vi "IR Opo Main.vi"() -> ()   [LabVIEW 2016] (continued)
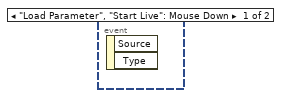
[diagram p2: hidden frame]
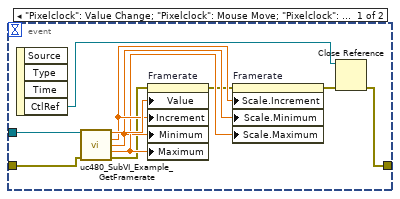
[diagram p3: hidden frame]
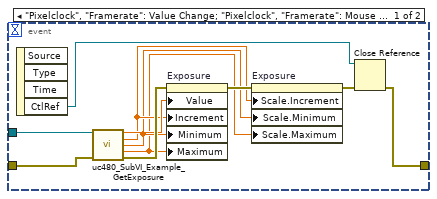
[diagram p4: hidden frame]
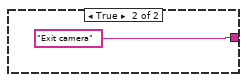
[diagram p5: hidden frame]
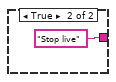
[diagram p6: hidden frame]
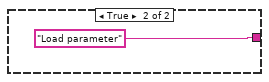
[diagram p7: hidden frame]
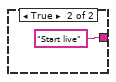
[diagram p8: hidden frame]
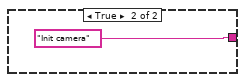
[diagram p9: hidden frame]
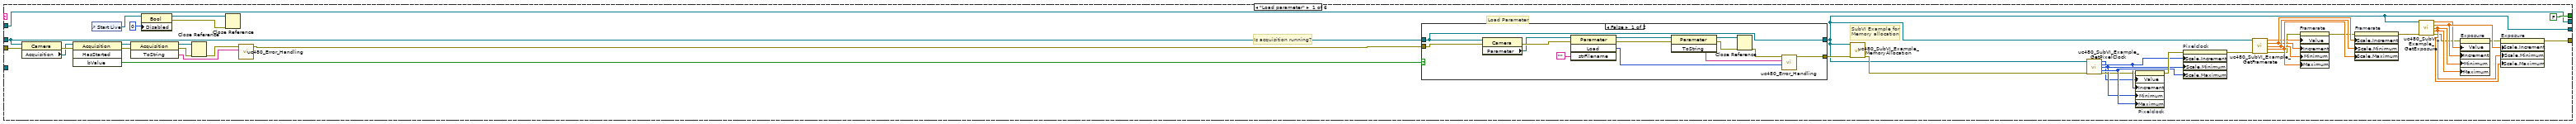
[diagram p10: hidden frame]
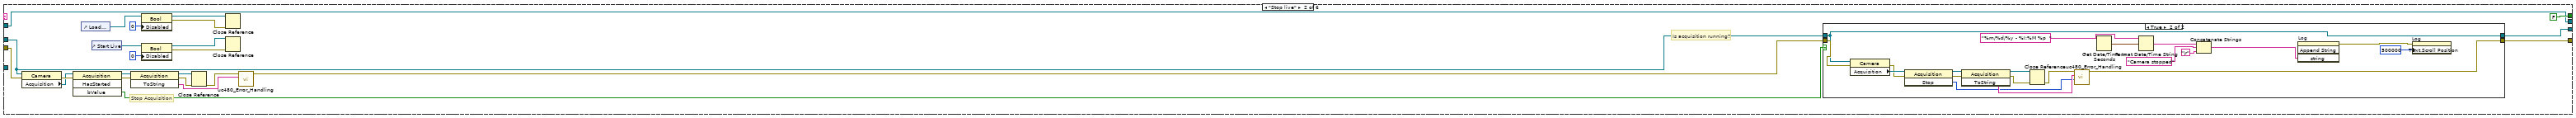
[diagram p12: hidden frame]
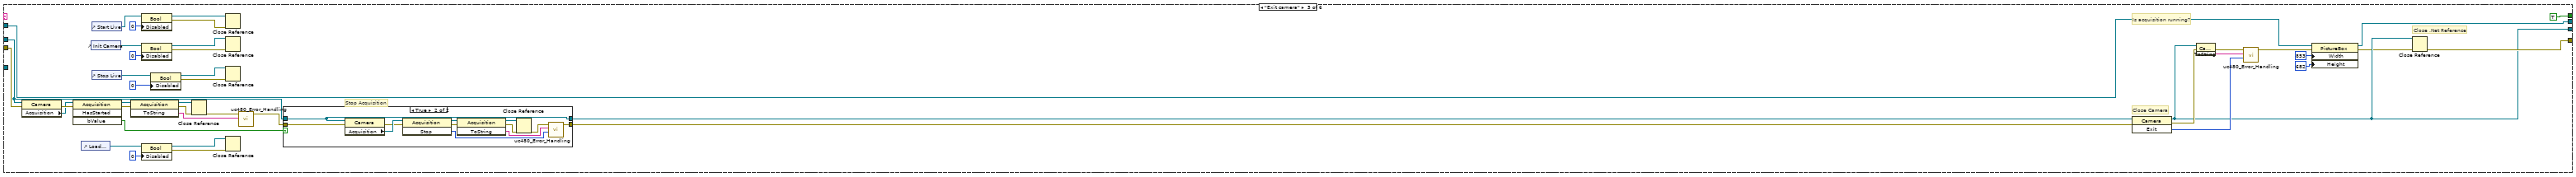
[diagram p14: hidden frame]
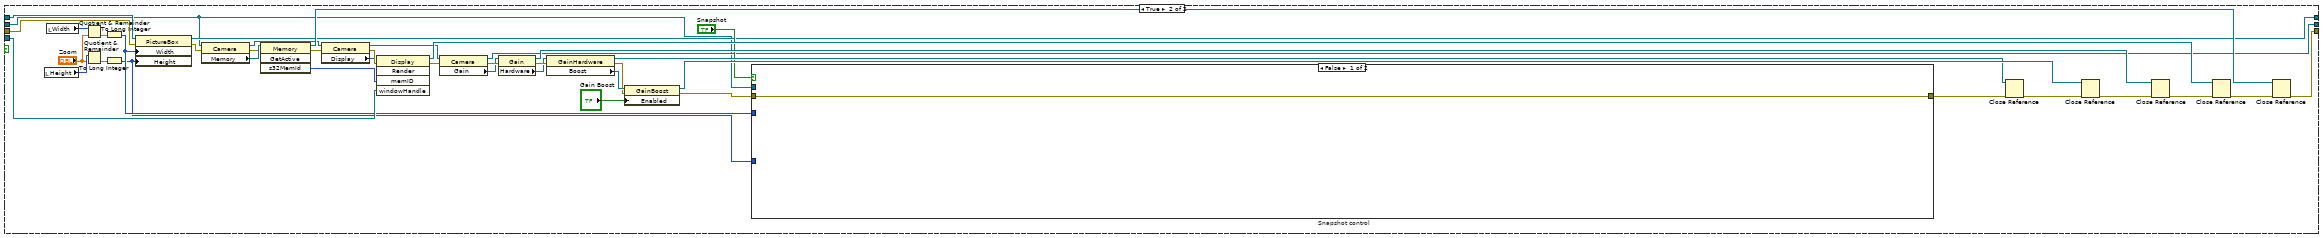
[diagram p16: hidden frame]
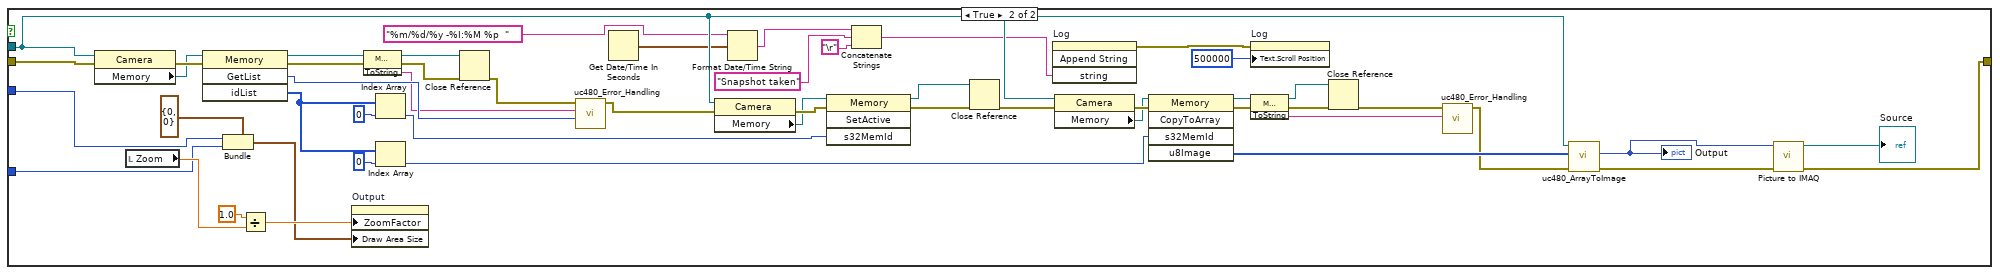
[diagram p17: hidden frame]
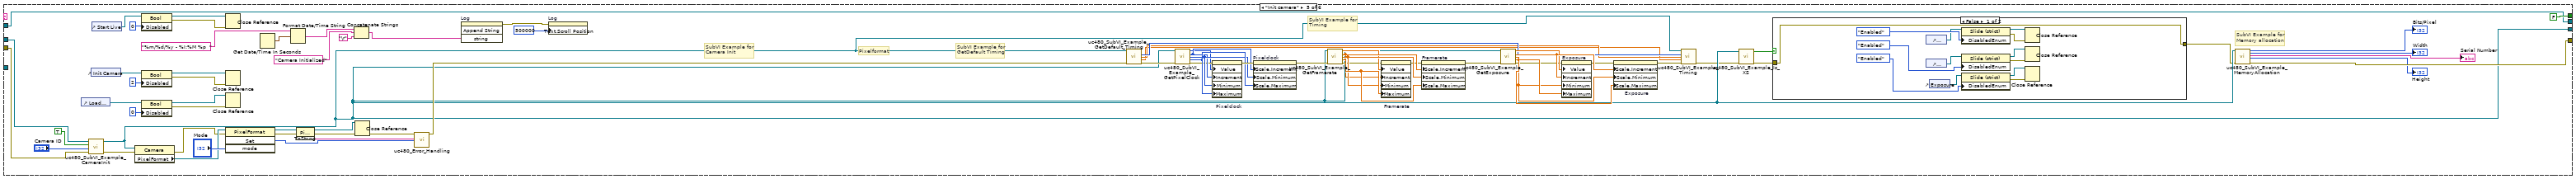
[diagram p18: hidden frame]
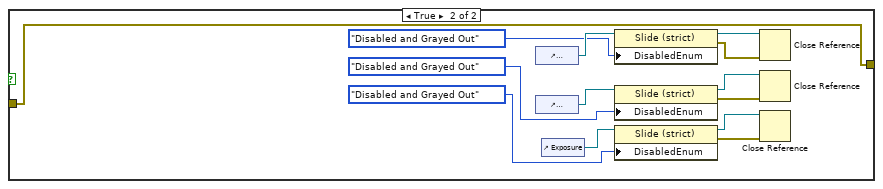
[diagram p19: hidden frame]
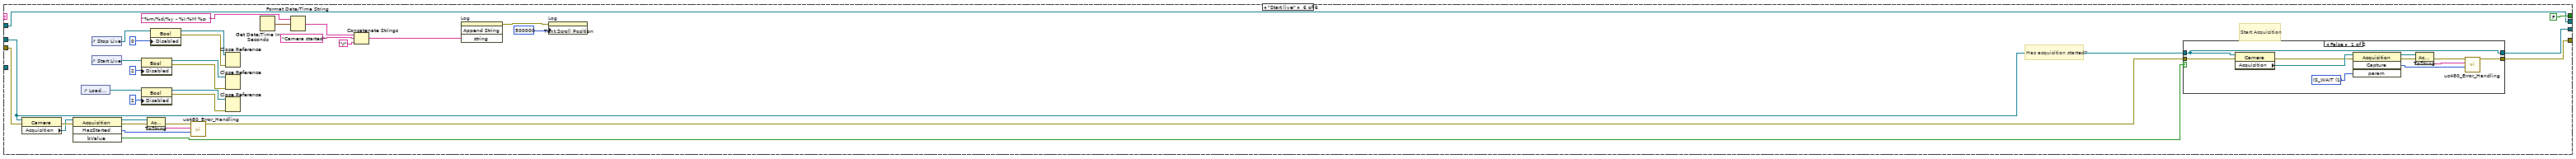
[diagram p20: hidden frame]
            n536 = local read "Y offset"() -> (w1451:i32)
            n537 = call <vilib>:"Simple Error Handler.vi"("error in (no error)"=w1382) -> ()  [unwired: 4 in, 5 out]
            n538 = Unbundle(w1387) -> ("Global Rectangle[0]"=w1386:i32, "Global Rectangle[1]"=w1385:i32)
            n539 = Empty Array?(array=w1437) -> (empty?=w1438:bool)
            n540 = Subtract(x=w1386, y=w1450) -> (x-y=w1457:i32)
            n541 = Subtract(x=w1385, y=w1451) -> (x-y=w1456:i32)
            n542 = case shown="False" w1438 {
              tunnel: [w1478 u8[][] [[1]] ("Image Pixels (U8)")] -> w1436
              tunnel: w1437 -> [w1478 _]
              frame False {
              }
              frame True {
                n543 = One Button Dialog(message="ATTENTION: you did not select\nany region of interest") -> ()  [unwired: 1 in, 1 out]
              }
            }
            n544 = local read "Heigth (µm)"() -> (w1421:i32)
            n545 = local read "Width (µm)"() -> (w1420:i32)
            n546 = Divide "X spot radius in micron"(x=w1420, y=w1415) -> (x/y=w1424:dbl)
            n547 = Divide "Y spot radius in micron"(x=w1421, y=w1415) -> (x/y=w1423:dbl)
            n548 = local read "Pixel size"() -> (w1389:dbl)
            n549 = Divide "X spot diameter in pixel"(x=w1420, y=w1389) -> (x/y=w1393:dbl)
            n550 = Divide "Y spot diameter in pixel"(x=w1421, y=w1389) -> (x/y=w1394:dbl)
            n551 = Multiply(x=w1389, y=w1389) -> (x*y=w1441:dbl)
            n552 = Multiply(x=w1457, y=w1389) -> (x*y=w1417:dbl)
            n553 = Multiply(x=w1456, y=w1389) -> (x*y=w1425:dbl)
            n554 = Round To Nearest(number=w1424) -> (nearest integer value=w1418:dbl)
            n555 = Round To Nearest(number=w1423) -> (nearest integer value=w1419:dbl)
            n556 = Add(x=w1417, y=w1418) -> (x+y=w1416:dbl)
            n557 = Add(x=w1425, y=w1419) -> (x+y=w1422:dbl)
            n558 = To Double Precision Float(number=w1436) -> (double precision float=w1439:dbl[][])
            n559 = Array Size(array=w1436) -> (size(s)=w1461:i32[])
            n560 = local read "Height  step \ndivider"() -> (w1463:i32)
            n561 = Divide(x=w1416, y=w1447) -> (x/y=w1449:dbl)
            n562 = Divide(x=w1422, y=w1447) -> (x/y=w1448:dbl)
            n563 = Add Array Elements(numeric array=w1439) -> (sum=w1443:dbl)
            n564 = Array To Cluster(array=w1461) -> (cluster=w1462:cluster{"[0]":i32, "[1]":i32})
            n565 = Number To Fractional String(number=w1449, precision (6)=w1455) -> (F-format string=w1434:string)  [unwired: 2 in]
            n566 = Number To Fractional String(number=w1448, precision (6)=w1455) -> (F-format string=w1435:string)  [unwired: 2 in]
            n567 = Unbundle(w1462) -> ("[0]"=w1381:i32, "[1]"=w1397:i32)
            n568 = Divide(x=w1443, y=u8 255) -> (x/y=w1440:dbl)
            n569 = Multiply "# pixels in an ablation spot"(x=w1394, y=w1393) -> (x*y=w1396:dbl)
            n570 = Multiply(x=w1440, y=w1441) -> (x*y=w1431:dbl)
            n571 = Multiply(x=w1381, y=w1389) -> (x*y=w1427:dbl)
            n572 = Multiply(x=w1397, y=w1389) -> (x*y=w1428:dbl)
            n573 = Subtract(x=w1397, y=w1393) -> (x-y=w1414:dbl)
            n574 = Fract/Exp String To Number(string=w1434) -> (number=→"Axis 1 Offset":dbl)  [unwired: 3 in, 1 out]
            n575 = Fract/Exp String To Number(string=w1435) -> (number=→"Axis 2 Offset":dbl)  [unwired: 3 in, 1 out]
            n576 = Divide "Height of a line"(x=w1394, y=w1463) -> (x/y=w1391:dbl)
            n577 = Divide "Total heigth lines"(x=w1381, y=w1391) -> (x/y=w1395:dbl)
            n578 = Multiply(x=w1389, y=w1391) -> (x*y=w1392:dbl)
            n579 = Round To Nearest(number=w1427) -> (nearest integer value=→"ROI container\nheigth (µm)":dbl)
            n580 = Round To Nearest(number=w1428) -> (nearest integer value=→"ROI container\nwidth (µm)":dbl)
            n581 = Divide(x=w1431, y=1000000.0) -> (x/y=→"ROI Area \n(mm2)":dbl)
            n582 = Divide(x="Precision (%)", y=100.0) -> (x/y=w1380:dbl)
            n583 = call "ROI parser.vi"("# pixels in an ablation spot"=w1396, "ROI Height in pixel"=w1395, "Heigth step size in pixel"=w1391, "ROI (8 bit image)"=w1436, "Ablation spot width"=w1393, "ROI Width in pixel"=w1414, "Sampling\nPrecision"=w1380, "Ablation spot heigth"=w1394) -> ("Parsed array"=w1476:bool[][])  [unwired: 3 in]
            n584 = Index Array(array=w1476, index (col)=0 ("disabled index (col)")) -> (element=w1474:bool[])  [unwired: 1 in]
            n585 = Array Size(array=w1474) -> (size(s)=w1475:i32)
            n586 = call "Array processor.vi"("Source array"=w1476, "Iterations"=w1475) -> ("Lenght product array"=w1473:i32[][], "T/F product array"=w1410:bool[][])  [unwired: 8 in]
            n587 = for {
              tunnel: w1473 -> [w1486] mode=indexing
              tunnel: [w1485] -> w1459 mode=indexing
              tunnel: w1389 -> [w1484]
              # "This loop transform each lenght fragment into a µm size value"
              n588 = Multiply(x=w1484, y=w1486) -> (x*y=w1485:dbl[])
            }
            n589 = Array Size(array=w1410) -> (size(s)=w1409:i32[])
            n590 = Index Array(array=w1410, index (col)=0 ("disabled index (col)")) -> (element=w1465:bool[])  [unwired: 1 in]
            n591 = Array Size(array=w1465) -> (size(s)=w1464:i32)
            n592 = Index Array(array=w1409, index=0) -> (element=w1406:i32)
            n593 = Index Array(array=w1409, index=1) -> (element=w1405:i32)
            n594 = for {
              N: w1464 -> [_]
              tunnel: w1410 -> [w1483] mode=indexing
              tunnel: [w1481] -> w1446 mode=indexing
              # "This loop add a F for each Y moviment"
              n595 = Build Array (concatenate)(w1483, FALSE) -> (w1481:bool[])
            }
            "Laser on/off array" <- w1446
            n596 = Multiply(x=w1406, y=w1405) -> (x*y=w1404:i32)
            n597 = Multiply(x=w1404, y=w1403) -> (x*y=w1402:dbl)
            n598 = Round To Nearest(number=w1392) -> (nearest integer value=w1390:dbl)
            n599 = local read "Speed (µm/s)"() -> (w1411:i32)
            n600 = Index Array(array=w1459, index (col)=0 ("disabled index (col)")) -> (element=w1469:dbl[])  [unwired: 1 in]
            n601 = Index Array(array=w1459, index (row)=0) -> (element=w1471:dbl[])  [unwired: 1 in]
            n602 = Array Size(array=w1469) -> (size(s)=w1467:i32)
            n603 = Array Size(array=w1471) -> (size(s)=w1470:i32)
            n604 = local read "Axis 1"() -> (w1413:string)
            n605 = local read "Axis 2"() -> (w1412:string)
            n606 = call "Commands array generator.vi"("Axis 1"=w1413, "Heigth"=w1467, "Axis in"=w1412, "Width"=w1470, "Axes speed \n(µm/s)"=w1411, "Y Step size in µm"=w1390, "T/F product array"=w1410, "Space defined array"=w1459) -> ("Command Array"=→"Commands array":string[][], "Time Array"=w1426:dbl[][])  [unwired: 2 in]
            "Time array" <- w1426
            n607 = Add Array Elements(numeric array=w1426) -> (sum=w1401:dbl)
            n608 = Add(x=w1402, y=w1401) -> (x+y=w1400:dbl)
            "Processi time (sec)" <- w1400
            n609 = local write "Process time"(w1400) -> ()
          }
        }
      }
      event "Axes Manual Control": Value Change {
        n610 = event-data() -> ()  [unwired: 1 in, 6 out]
        n611 = case shown="True" "Axes Manual Control" {
          tunnel: w1489 -> [_ w1501]
          tunnel: w1488 -> [_ w1500]
          tunnel: w1487 -> [_ w1499]
          frame False {
          }
          frame True {
            n612 = flat-sequence {
              tunnel: w1501 -> [w1511]
              tunnel: w1500 -> [w1510]
              tunnel: w1499 -> [w1509]
              tunnel: [w1511] -> w1498
              tunnel: [w1510] -> w1497
              tunnel: [w1509] -> w1496
              tunnel: [w1508] -> w1495
              tunnel: [w1507] -> w1494
              tunnel: [w1506] -> w1493
              tunnel: [w1505] -> w1492
              tunnel: w1498 -> [w1554]
              tunnel: w1497 -> [w1553]
              tunnel: w1496 -> [w1552]
              tunnel: w1495 -> [w1547]
              tunnel: w1494 -> [w1546]
              tunnel: w1493 -> [w1537]
              tunnel: w1492 -> [w1536]
              frame #0 {
                n613 = call <userlib>:"Open TCP-IP.vi"("IP address"=w1511) -> ("error out"=w1503:errorcluster, "Connection ID"=w1512:T6)  [unwired: 8 in, 1 out]
                n614 = call <vilib>:"Simple Error Handler.vi"("error in (no error)"=w1503) -> ("error?"=w1502:bool, "error out"=w1504:errorcluster)  [unwired: 4 in, 3 out]
                n615 = case shown="True" w1502 {
                  tunnel: w1512 -> [w1527 _]
                  tunnel: w1504 -> [w1526 _]
                  tunnel: w1510 -> [w1523 _]
                  tunnel: w1509 -> [w1522 _]
                  tunnel: [w1521 w1531] -> w1508
                  tunnel: [w1520 w1531] -> w1507
                  tunnel: [w1516 w1530] -> w1506
                  tunnel: [w1515 w1530] -> w1505
                  frame False {
                    n616 = call "Get Stages Status.vi"("error in (no error)"=w1526, "Group Name (250 c max)"=w1523, "connection ID in"=w1527) -> ("error out"=w1525:errorcluster, "XPS error out"=w1524:errorcluster, "Group Status String"=w1520:string, "connection ID out"=w1519:T6, "Status"=w1515:i32)  [unwired: 4 in]
                    n617 = call "Get Stages Status.vi"("error in (no error)"=w1525, "XPS error in (no error)"=w1524, "Group Name (250 c max)"=w1522, "connection ID in"=w1519) -> ("error out"=w1529:errorcluster, "XPS error out"=w1518:errorcluster, "Group Status String"=w1521:string, "connection ID out"=w1528:T6, "Status"=w1516:i32)  [unwired: 3 in]
                    n618 = call <vilib>:"Simple Error Handler.vi"("error source (\" \")"="Axis manual control check" ("error source (\" \")"), "error in (no error)"=w1518) -> ()  [unwired: 3 in, 5 out]
                    n619 = call <userlib>:"Close TCP-IP.vi"("error in (no error)"=w1529, "connection ID in"=w1528) -> ("Error out"=w1517:errorcluster)  [unwired: 9 in]
                    n620 = call <vilib>:"Simple Error Handler.vi"("error source (\" \")"="TCP close Axis manual control check" ("error source (\" \")"), "error in (no error)"=w1517) -> ()  [unwired: 3 in, 5 out]
                  }
                  frame True {
                    w1530 = 0
                    w1531 = ""
                  }
                }
              }
              frame #1 {
                w1540 = 47 ("y")
                w1541 = "Ready"
                n621 = String Subset(string=w1546, offset (0)=0, length (rest)=5 ("length (rest)")) -> (substring=w1543:string)
                n622 = String Subset(string=w1547, offset (0)=0, length (rest)=5 ("length (rest)")) -> (substring=w1542:string)
                n623 = Equal?(x=w1543, y=w1541) -> (x = y?=w1544:bool)
                n624 = Equal?(x=w1541, y=w1542) -> (x = y?=w1545:bool)
                n625 = Equal?(x=w1540, y=w1536) -> (x = y?=w1538:bool)
                n626 = Equal?(x=w1537, y=w1540) -> (x = y?=w1539:bool)
                n627 = And(x=w1539, y=w1538) -> (x .and. y?=w1533:bool)
                n628 = And(x=w1544, y=w1545) -> (x .and. y?=w1534:bool)
                n629 = Not(x=w1533) -> (.not. x?=w1532:bool)
                n630 = And(x=w1534, y=w1532) -> (x .and. y?=w1535:bool)
                n631 = case shown="True" w1535 {
                  tunnel: w1554 -> [_ w1560]
                  tunnel: w1553 -> [_ w1559]
                  tunnel: w1552 -> [_ w1558]
                  tunnel: w1532 -> [w1555 _]
                  frame False {
                    n632 = case shown="False" w1555 {
                      frame False {
                        n633 = One Button Dialog(message="One or more axis already in jogging position") -> ()  [unwired: 1 in, 1 out]
                      }
                      frame True {
                        n634 = One Button Dialog(message="Axes are not ready") -> ()  [unwired: 1 in, 1 out]
                      }
                    }
                  }
                  frame True {
                    n635 = call "XPS_LTA_HS_Jogger.vi"("Axis 2"=w1558, "Axis 1"=w1559, "Controller Address"=w1560) -> ()  [unwired: 8 in]
                  }
                }
              }
            }
          }
        }
      }
      event "Home Axes": Value Change {
        n636 = event-data() -> ()  [unwired: 1 in, 6 out]
        n637 = flat-sequence {
          tunnel: w1567 -> [w1573]
          tunnel: w1568 -> [w1574]
          tunnel: w1569 -> [w1575]
          tunnel: "Home Axes" -> [w1576]
          tunnel: [w1576] -> w1565
          tunnel: [w1575] -> w1564
          tunnel: [w1574] -> w1563
          tunnel: [w1573] -> w1562
          tunnel: [w1572] -> w1561
          tunnel: [w1580] -> w1566
          tunnel: w1565 -> [w1578]
          tunnel: w1564 -> [w1583]
          tunnel: w1563 -> [w1581]
          tunnel: w1562 -> [w1582]
          tunnel: w1561 -> [w1579]
          tunnel: [w1662] -> w1570
          tunnel: w1566 -> [w1661]
          frame #0 {
            n638 = call "Display Message to User"() -> ("OK"=w1572:bool)  [unwired: 10 in, 1 out]
          }
          frame #1 {
            n639 = And(x=w1578, y=w1579) -> (x .and. y?=w1577:bool)
            n640 = case shown="True" w1577 {
              tunnel: w1583 -> [_ w1599]
              tunnel: w1581 -> [_ w1600]
              tunnel: w1582 -> [_ w1597]
              tunnel: w1581 -> [_ w1598]
              tunnel: [FALSE w1590] -> w1580
              frame False {
              }
              frame True {
                w1596 = 47 ("y")
                w1612 = "Ready"
                n641 = call <userlib>:"Open TCP-IP.vi"("IP address"=w1599) -> ("error out"=w1585:errorcluster, "Connection ID"=w1603:T6)  [unwired: 8 in, 1 out]
                n642 = call <vilib>:"Simple Error Handler.vi"("error in (no error)"=w1585) -> ("error?"=w1587:bool, "error out"=w1586:errorcluster)  [unwired: 4 in, 3 out]
                n643 = case shown="True" w1587 {
                  tunnel: w1586 -> [w1626 _]
                  tunnel: w1603 -> [w1625 _]
                  tunnel: [w1622 w1631] -> w1602
                  tunnel: [w1621 w1631] -> w1601
                  tunnel: w1600 -> [w1620 _]
                  tunnel: w1597 -> [w1619 _]
                  tunnel: [w1616 w1630] -> w1595
                  tunnel: [w1615 w1630] -> w1594
                  frame False {
                    n644 = call "Get Stages Status.vi"("error in (no error)"=w1626, "Group Name (250 c max)"=w1620, "connection ID in"=w1625) -> ("error out"=w1627:errorcluster, "XPS error out"=w1628:errorcluster, "Group Status String"=w1622:string, "connection ID out"=w1629:T6, "Status"=w1615:i32)  [unwired: 4 in]
                    n645 = call "Get Stages Status.vi"("error in (no error)"=w1627, "XPS error in (no error)"=w1628, "Group Name (250 c max)"=w1619, "connection ID in"=w1629) -> ("error out"=w1623:errorcluster, "XPS error out"=w1618:errorcluster, "Group Status String"=w1621:string, "connection ID out"=w1624:T6, "Status"=w1616:i32)  [unwired: 3 in]
                    n646 = call <vilib>:"Simple Error Handler.vi"("error source (\" \")"="home axis check" ("error source (\" \")"), "error in (no error)"=w1618) -> ()  [unwired: 3 in, 5 out]
                    n647 = call <userlib>:"Close TCP-IP.vi"("error in (no error)"=w1623, "connection ID in"=w1624) -> ("Error out"=w1617:errorcluster)  [unwired: 9 in]
                    n648 = call <vilib>:"Simple Error Handler.vi"("error source (\" \")"="TCP close home axis check" ("error source (\" \")"), "error in (no error)"=w1617) -> ()  [unwired: 3 in, 5 out]
                  }
                  frame True {
                    w1630 = 0
                    w1631 = ""
                  }
                }
                n649 = Equal?(x=w1596, y=w1594) -> (x = y?=w1593:bool)
                n650 = Equal?(x=w1595, y=w1596) -> (x = y?=w1592:bool)
                n651 = String Subset(string=w1602, offset (0)=0, length (rest)=5 ("length (rest)")) -> (substring=w1610:string)
                n652 = String Subset(string=w1601, offset (0)=0, length (rest)=5 ("length (rest)")) -> (substring=w1611:string)
                n653 = Equal?(x=w1610, y=w1612) -> (x = y?=w1609:bool)
                n654 = Equal?(x=w1612, y=w1611) -> (x = y?=w1608:bool)
                n655 = And(x=w1592, y=w1593) -> (x .and. y?=w1588:bool)
                n656 = Not(x=w1588) -> (.not. x?=w1589:bool)
                n657 = And(x=w1609, y=w1608) -> (x .and. y?=w1591:bool)
                n658 = And(x=w1591, y=w1589) -> (x .and. y?=w1590:bool)
                n659 = case shown="True" w1590 {
                  tunnel: w1599 -> [_ w1641]
                  tunnel: w1598 -> [_ w1640]
                  tunnel: w1597 -> [_ w1639]
                  tunnel: w1588 -> [w1632 _]
                  frame False {
                    n660 = case shown="True" w1632 {
                      frame False {
                        n661 = One Button Dialog(message="Axes are not ready") -> ()  [unwired: 1 in, 1 out]
                      }
                      frame True {
                        n662 = One Button Dialog(message="One or more axis are in jogging mode") -> ()  [unwired: 1 in, 1 out]
                      }
                    }
                  }
                  frame True {
                    n663 = call <userlib>:"Open TCP-IP.vi"("IP address"=w1641) -> ("error out"=w1657:errorcluster, "Connection ID"=w1658:T6)  [unwired: 8 in, 1 out]
                    n664 = call <userlib>:"Group Kill.vi"("error in (no error)"=w1657, "Group Name (250 c max)"=w1640, "connection ID in"=w1658) -> ("error out"=w1655:errorcluster, "XPS error out"=w1656:errorcluster, "connection ID out"=w1652:T6)  [unwired: 6 in]
                    n665 = call <userlib>:"Group Initialize.vi"("error in (no error)"=w1655, "XPS error in (no error)"=w1656, "Group Name (250 c max)"=w1640, "connection ID in"=w1652) -> ("error out"=w1653:errorcluster, "XPS error out"=w1654:errorcluster, "connection ID out"=w1651:T6)  [unwired: 5 in]
                    n666 = call <userlib>:"Group Home Search.vi"("error in (no error)"=w1653, "XPS error in (no error)"=w1654, "Group Name (250 c max)"=w1640, "connection ID in"=w1651) -> ("error out"=w1642:errorcluster, "XPS error out"=w1643:errorcluster, "connection ID out"=w1650:T6)  [unwired: 5 in]
                    n667 = call <userlib>:"Group Kill.vi"("error in (no error)"=w1642, "XPS error in (no error)"=w1643, "Group Name (250 c max)"=w1639, "connection ID in"=w1650) -> ("error out"=w1644:errorcluster, "XPS error out"=w1645:errorcluster, "connection ID out"=w1649:T6)  [unwired: 5 in]
                    n668 = call <userlib>:"Group Initialize.vi"("error in (no error)"=w1644, "XPS error in (no error)"=w1645, "Group Name (250 c max)"=w1639, "connection ID in"=w1649) -> ("error out"=w1646:errorcluster, "XPS error out"=w1647:errorcluster, "connection ID out"=w1648:T6)  [unwired: 5 in]
                    n669 = call <userlib>:"Group Home Search.vi"("error in (no error)"=w1646, "XPS error in (no error)"=w1647, "Group Name (250 c max)"=w1639, "connection ID in"=w1648) -> ("error out"=w1659:errorcluster, "XPS error out"=w1638:errorcluster, "connection ID out"=w1660:T6)  [unwired: 5 in]
                    n670 = call <vilib>:"Simple Error Handler.vi"("error source (\" \")"="home axis " ("error source (\" \")"), "error in (no error)"=w1638) -> ()  [unwired: 3 in, 5 out]
                    n671 = call <userlib>:"Close TCP-IP.vi"("error in (no error)"=w1659, "connection ID in"=w1660) -> ("Error out"=w1637:errorcluster)  [unwired: 9 in]
                    n672 = call <vilib>:"Simple Error Handler.vi"("error source (\" \")"="TCP close home axis " ("error source (\" \")"), "error in (no error)"=w1637) -> ()  [unwired: 3 in, 5 out]
                  }
                }
              }
            }
          }
          frame #2 {
            n673 = case shown="True" w1661 {
              tunnel: ["" ("StringOut") "Axes have been moved to home position" ("StringOut")] -> w1662
              frame False {
              }
              frame True {
              }
            }
          }
        }
      }
      event "Transparency": Value Change {
        n674 = event-data() -> ()  [unwired: 1 in, 6 out]
        n675 = control-ref of="This VI"() -> (w1666:refnum<vi>)
        n676 = property class="VI"(reference=w1666, "FP:Transparency"="Transparency") -> ()  [unwired: 1 in, 2 out]
      }
      event "Capture": Value Change {
        w1677 = 47 ("y")
        w1693 = "Ready"
        n677 = event-data() -> ()  [unwired: 1 in, 6 out]
        n678 = call <userlib>:"Open TCP-IP.vi"("IP address"=w1681) -> ("error out"=w1669:errorcluster, "Connection ID"=w1684:T6)  [unwired: 8 in, 1 out]
        n679 = call <vilib>:"Simple Error Handler.vi"("error in (no error)"=w1669) -> ("error?"=w1667:bool, "error out"=w1668:errorcluster)  [unwired: 4 in, 3 out]
        n680 = case shown="True" w1667 {
          tunnel: w1668 -> [w1707 _]
          tunnel: w1684 -> [w1706 _]
          tunnel: [w1703 w1711] -> w1683
          tunnel: [w1702 w1711] -> w1682
          tunnel: w1680 -> [w1701 _]
          tunnel: w1679 -> [w1700 _]
          tunnel: [w1698 w1712] -> w1678
          tunnel: [w1697 w1712] -> w1676
          frame False {
            n681 = call "Get Stages Status.vi"("error in (no error)"=w1707, "Group Name (250 c max)"=w1701, "connection ID in"=w1706) -> ("error out"=w1708:errorcluster, "XPS error out"=w1709:errorcluster, "Group Status String"=w1703:string, "connection ID out"=w1710:T6, "Status"=w1697:i32)  [unwired: 4 in]
            n682 = call "Get Stages Status.vi"("error in (no error)"=w1708, "XPS error in (no error)"=w1709, "Group Name (250 c max)"=w1700, "connection ID in"=w1710) -> ("error out"=w1704:errorcluster, "XPS error out"=w1699:errorcluster, "Group Status String"=w1702:string, "connection ID out"=w1705:T6, "Status"=w1698:i32)  [unwired: 3 in]
            n683 = call <vilib>:"Simple Error Handler.vi"("error source (\" \")"="Capture check" ("error source (\" \")"), "error in (no error)"=w1699) -> ()  [unwired: 3 in, 5 out]
            n684 = call <userlib>:"Close TCP-IP.vi"("error in (no error)"=w1704, "connection ID in"=w1705) -> ("Error out"=w1695:errorcluster)  [unwired: 9 in]
            n685 = call <vilib>:"Simple Error Handler.vi"("error in (no error)"=w1695) -> ()  [unwired: 4 in, 5 out]
          }
          frame True {
            w1712 = 0
            w1711 = ""
          }
        }
        n686 = Equal?(x=w1677, y=w1676) -> (x = y?=w1674:bool)
        n687 = Equal?(x=w1678, y=w1677) -> (x = y?=w1675:bool)
        n688 = String Subset(string=w1683, offset (0)=0, length (rest)=5 ("length (rest)")) -> (substring=w1691:string)
        n689 = String Subset(string=w1682, offset (0)=0, length (rest)=5 ("length (rest)")) -> (substring=w1692:string)
        n690 = Equal?(x=w1691, y=w1693) -> (x = y?=w1690:bool)
        n691 = Equal?(x=w1693, y=w1692) -> (x = y?=w1689:bool)
        n692 = And(x=w1675, y=w1674) -> (x .and. y?=w1671:bool)
        n693 = And(x=w1690, y=w1689) -> (x .and. y?=w1673:bool)
        n694 = Not(x=w1671) -> (.not. x?=w1670:bool)
        n695 = And(x=w1673, y=w1670) -> (x .and. y?=w1672:bool)
        n696 = case shown="True" w1672 {
          tunnel: ["" w1720] -> w1694
          tunnel: w1681 -> [_ w1719]
          tunnel: w1679 -> [_ w1718]
          tunnel: w1680 -> [_ w1717]
          tunnel: w1671 -> [w1713 _]
          frame False {
            n697 = case shown="True" w1713 {
              frame False {
                n698 = One Button Dialog(message="Axes are not ready") -> ()  [unwired: 1 in, 1 out]
              }
              frame True {
                n699 = One Button Dialog(message="One or more axis are in jogging mode") -> ()  [unwired: 1 in, 1 out]
              }
            }
          }
          frame True {
            n700 = flat-sequence {
              tunnel: [w1741] -> w1732
              tunnel: [w1740] -> w1731
              tunnel: [w1739] -> w1730
              tunnel: [w1738] -> w1729
              tunnel: [w1737] -> w1728
              tunnel: [w1736] -> w1727
              tunnel: [w1735] -> w1726
              tunnel: w1719 -> [w1735]
              tunnel: w1718 -> [w1734]
              tunnel: w1717 -> [w1733]
              tunnel: w1732 -> [w1761]
              tunnel: w1731 -> [w1752]
              tunnel: w1730 -> [w1753]
              tunnel: w1729 -> [w1759]
              tunnel: w1728 -> [w1758]
              tunnel: [w1751] -> w1725
              tunnel: w1727 -> [w1751]
              tunnel: [w1750] -> w1724
              tunnel: w1726 -> [w1750]
              tunnel: [w1763] -> w1723
              tunnel: w1725 -> [w1763]
              tunnel: [w1762] -> w1722
              tunnel: w1724 -> [w1762]
              tunnel: w1723 -> [w1771]
              tunnel: w1722 -> [w1776]
              tunnel: [w1770] -> w1721
              tunnel: [w1785] -> w1720
              tunnel: w1721 -> [w1782]
              frame #0 {
                w1746 = ".Pos"
                n701 = local read "Axis Initial Parameters"() -> (w1736:T1)
                n702 = Concatenate Strings(w1733, w1746) -> (w1740:string)
                n703 = call <userlib>:"Open TCP-IP.vi"("IP address"=w1735) -> ("error out"=w1742:errorcluster, "Connection ID"=w1747:T6)  [unwired: 5 in, 4 out]
                n704 = call <userlib>:"Positioner SGamma Parameters Set.vi"("SGamma Parameters"=w1736, "error in (no error)"=w1742, "Positioner Name (250 c max)"=w1740, "connection ID in"=w1747) -> ("error out"=w1743:errorcluster, "XPS error out"=w1744:errorcluster, "connection ID out"=w1745:T6)  [unwired: 5 in]
                n705 = Concatenate Strings(w1734, w1746) -> (w1739:string)
                n706 = call <userlib>:"Positioner SGamma Parameters Set.vi"("SGamma Parameters"=w1736, "error in (no error)"=w1743, "XPS error in (no error)"=w1744, "Positioner Name (250 c max)"=w1739, "connection ID in"=w1745) -> ("error out"=w1738:errorcluster, "XPS error out"=w1737:errorcluster, "connection ID out"=w1741:T6)  [unwired: 4 in]
              }
              frame #1 {
                n707 = local read "Axis 2 Offset"() -> (w1749:dbl)
                n708 = local read "Axis 1 Offset"() -> (w1748:dbl)
                n709 = call <userlib>:"Single Axis Group Move Relative.vi"("Target Displacement (units)"=w1749, "error in (no error)"=w1759, "XPS error in (no error)"=w1758, "SingleAxis Group  Name (250 c max)"=w1752, "connection ID in"=w1761) -> ("error out"=w1756:errorcluster, "XPS error out"=w1757:errorcluster, "connection ID out"=w1760:T6)  [unwired: 4 in]
                n710 = call <userlib>:"Single Axis Group Move Relative.vi"("Target Displacement (units)"=w1748, "error in (no error)"=w1756, "XPS error in (no error)"=w1757, "SingleAxis Group  Name (250 c max)"=w1753, "connection ID in"=w1760) -> ("error out"=w1754:errorcluster, "connection ID out"=w1755:T6)  [unwired: 4 in, 1 out]
                n711 = call <userlib>:"Close TCP-IP.vi"("error in (no error)"=w1754, "connection ID in"=w1755) -> ()  [unwired: 9 in, 1 out]
              }
              frame #2 {
                n712 = Wait (ms)(milliseconds to wait=u32 1000) -> ()  [unwired: 1 out]
              }
              frame #3 {
                n713 = local read "Speed (µm/s)"() -> (w1775:i32)
                n714 = local read "Processi time (sec)"() -> (w1769:i32)
                n715 = local read "Laser on/off array"() -> (w1779:bool[][])
                n716 = local read "Commands array"() -> (w1780:string[][])
                n717 = local read "ROI Area \n(mm2)"() -> (w1767:dbl)
                n718 = Divide(x=w1775, y=1000) -> (x/y=w1772:dbl)
                n719 = local read "VISA Laser port"() -> (w1765:string)
                n720 = local read "Laser Com Delay"() -> (w1766:i32)
                n721 = call "IR_OPO_Capture_V2.vi"("Commands array"=w1780, "XPS_Address"=w1776, "VISA resource name"=w1765, "laser array index"=0, "Process time"=w1769, "Axis Speed"=w1772, "Laser on/off array"=w1779, "stop"=FALSE ("STOP CAPTURE"), "delay before read (ms)"=w1766, "Axis Initial Parameters"=w1771, "ROI Area \n(mm2)"=w1767, "OPO on?"=TRUE, "Acceleration (units/seconds²)"="Acceleration \n(mm/s²)") -> ("Elapsed time"=w1770:dbl)  [unwired: 6 in]
              }
              frame #4 {
                n722 = Number To Decimal String(number=w1782) -> (decimal integer string=w1781:string)  [unwired: 1 in]
                n723 = Concatenate Strings("Capture completed in " ("StringOut"), w1781, " seconds" ("string")) -> (w1785:string)
              }
            }
          }
        }
      }
    }
    n724 = Get Date/Time In Seconds() -> (seconds since 1Jan1904=w856:timestamp)
    n725 = Format Date/Time String(time format string (%c)="%m/%d/%y - %I:%M %p  ", seconds (now)=w856) -> (date/time string=w855:string)  [unwired: 1 in]
    n726 = Empty String/Path?(string/path=w852) -> (empty?=w854:bool)
    n727 = Concatenate Strings(w855, w852, "\r") -> (w853:string)
    n728 = case shown="False" w854 {
      tunnel: w853 -> [w862 _]
      frame False {
        n729 = invoke on="Log" class="Str" method="Append String"("string"=w862) -> (error out=w861:errorcluster)  [unwired: 3 in, 3 out]
        n730 = property on="Log" class="Str"(error in=w861, "Text.Scroll Position"=u32 500000) -> ()  [unwired: 1 in, 2 out]
      }
      frame True {
      }
    }
  }
  n731 = control-ref of="Init Camera"() -> (w45:refnum<vi>)
  n732 = control-ref of="Stop Live"() -> (w38:refnum<vi>)
  n733 = property class="Bool"(reference=w38, "Disabled"=u8 2 ("Deaktiviert")) -> (reference out=w29:refnum<vi>, error out=w28:errorcluster)  [unwired: 1 in]
  n734 = property class="Bool"(reference=w45, "Disabled"=u8 0 ("Deaktiviert")) -> (reference out=w33:refnum<vi>, error out=w32:errorcluster)  [unwired: 1 in]
  n735 = Close Reference(reference=w29, error in (no error)=w28) -> ()  [unwired: 1 out]
  n736 = Close Reference(reference=w33, error in (no error)=w32) -> ()  [unwired: 1 out]
  n737 = control-ref of="Load Parameter"() -> (w39:refnum<vi>)
  n738 = control-ref of="Start Live"() -> (w42:refnum<vi>)
  n739 = property class="Bool"(reference=w42, "Disabled"=u8 2 ("Deaktiviert")) -> (reference out=w31:refnum<vi>, error out=w30:errorcluster)  [unwired: 1 in]
  n740 = property class="Bool"(reference=w39, "Disabled"=u8 2 ("Deaktiviert")) -> (reference out=w27:refnum<vi>, error out=w26:errorcluster)  [unwired: 1 in]
  n741 = Close Reference(reference=w31, error in (no error)=w30) -> ()  [unwired: 1 out]
  n742 = Close Reference(reference=w27, error in (no error)=w26) -> ()  [unwired: 1 out]
